vi "UHR-Fleezers Control (host) - Avogadro v1.vi"() -> ()   [LabVIEW 2014] (continued)
          }
          frame True {
          }
        }
        n2943 = local write "Tab Control 6"(T57."Imaging" ("Tab Control 6")) -> ()
        n2944 = local read "T3 X (V)"() -> (w5126:dbl)
        n2945 = local write "MCL Scanning"(w5134) -> ()
        n2946 = local read "T3 Y (V)"() -> (w5125:dbl)
        n2947 = local read "AO2"() -> (w5127:dbl)
        n2948 = local read "AO1"() -> (w5128:dbl)
        n2949 = case shown="True" "Center Scan" {
          tunnel: w5139 -> [w5157 w5179]
          tunnel: w5138 -> [w5156 w5178]
          tunnel: [w5155 w5177] -> w5136
          tunnel: [w5154 w5176] -> w5135
          tunnel: [w5149 w5173] -> w5133
          tunnel: [w5150 w5172] -> w5132
          tunnel: w5128 -> [w5147 w5175]
          tunnel: w5127 -> [w5146 w5174]
          tunnel: "Scan trap 3 or Fl?" -> [w5152 w5171]
          tunnel: w5126 -> [w5151 w5164]
          tunnel: w5125 -> [w5148 w5165]
          frame False {
            w5153 = TRUE ("AI to FIFO")
            n2950 = case shown="True" w5152 {
              tunnel: [w5159 w5163] -> w5150
              tunnel: w5151 -> [_ w5163]
              tunnel: [w5160 w5162] -> w5149
              tunnel: w5148 -> [_ w5162]
              tunnel: w5147 -> [w5160 _]
              tunnel: w5146 -> [w5159 _]
              tunnel: [FALSE ("AI to FIFO") TRUE ("AI to FIFO")] -> w5145
              frame False {
              }
              frame True {
              }
            }
            n2951 = xnode "Read/Write Control"("FPGA VI Reference In"=w5157, "error in"=w5156, "AI to FIFO"=w5153, "APD to FIFO"=w5153, "Start scan (MCL)"=w5153, "ScanTrap 3 or Fl-laser"=w5145) -> ("FPGA VI Reference Out"=w5155:T41, "error out"=w5154:errorcluster)
          }
          frame True {
            n2952 = local read "Actual MCL Inc (V)"() -> (w5166:dbl)
            n2953 = local read "Scan steps (MCL)"() -> (w5167:u64)
            n2954 = local read "Scan lines (y)"() -> (w5168:u64)
            n2955 = local read "Fast Scan Dir"() -> (w5169:bool)
            n2956 = local read "2D or 1D Scan"() -> (w5170:bool)
            n2957 = case shown="True" w5171 {
              tunnel: w5179 -> [w5197 w5215]
              tunnel: w5178 -> [w5196 w5214]
              tunnel: [w5195 w5213] -> w5177
              tunnel: [w5194 w5212] -> w5176
              tunnel: w5175 -> [w5190 _]
              tunnel: w5174 -> [w5189 _]
              tunnel: [w5187 w5207] -> w5173
              tunnel: [w5186 w5206] -> w5172
              tunnel: w5170 -> [w5185 w5205]
              tunnel: w5169 -> [w5184 w5204]
              tunnel: w5168 -> [w5183 w5203]
              tunnel: w5167 -> [w5182 w5202]
              tunnel: w5166 -> [w5180 w5200]
              tunnel: w5165 -> [_ w5199]
              tunnel: w5164 -> [_ w5198]
              frame False {
                w5193 = TRUE ("AI to FIFO")
                n2958 = Bundle("Actual MCL Inc (V)"=w5180, "Scan steps (MCL)"=w5182, "Scan lines (y)"=w5183, "AO1"=w5190, "AO2"=w5189) -> (w5188:T61)  [unwired: 1 in]
                n2959 = call "Center Scan calculation.vi"("2D or 1D Scan"=w5185, "Fast Scan Dir"=w5184, "Input parameters"=w5188) -> ("X"=w5186:dbl, "Y"=w5187:dbl)
                n2960 = call "Volt to I16.vi"("Voltage In"=w5187) -> ("I16 Voltage Out"=w5192:i16)
                n2961 = call "Volt to I16.vi"("Voltage In"=w5186) -> ("I16 Voltage Out"=w5191:i16)
                n2962 = xnode "Read/Write Control"("FPGA VI Reference In"=w5197, "error in"=w5196, "AI to FIFO"=w5193, "APD to FIFO"=w5193, "Start scan (MCL)"=w5193, "AO1 (Y)"=w5192, "AO2 (X)"=w5191, "ScanTrap 3 or Fl-laser"=FALSE ("AI to FIFO")) -> ("FPGA VI Reference Out"=w5195:T41, "error out"=w5194:errorcluster)
              }
              frame True {
                w5211 = TRUE ("AI to FIFO")
                n2963 = Bundle("Actual MCL Inc (V)"=w5200, "Scan steps (MCL)"=w5202, "Scan lines (y)"=w5203, "T3 Y (V)"=w5199, "T3 X (V)"=w5198) -> (w5208:T62)  [unwired: 1 in]
                n2964 = call "Center Scan calculation.vi"("2D or 1D Scan"=w5205, "Fast Scan Dir"=w5204, "Input parameters"=w5208) -> ("X"=w5206:dbl, "Y"=w5207:dbl)
                n2965 = call "Volt to I16.vi"("Voltage In"=w5207) -> ("I16 Voltage Out"=w5210:i16)
                n2966 = call "Volt to I16.vi"("Voltage In"=w5206) -> ("I16 Voltage Out"=w5209:i16)
                n2967 = xnode "Read/Write Control"("FPGA VI Reference In"=w5215, "error in"=w5214, "AI to FIFO"=w5211, "APD to FIFO"=w5211, "Start scan (MCL)"=w5211, "Piezo Trap Y (AO4)"=w5210, "Piezo Trap X (AO5)"=w5209, "ScanTrap 3 or Fl-laser"=TRUE ("AI to FIFO")) -> ("FPGA VI Reference Out"=w5213:T41, "error out"=w5212:errorcluster)
              }
            }
          }
        }
        "Initial Y" <- w5133
        "Initial X" <- w5132
        "wait to reset values" <- w5134
      }
    }
    n2968 = xnode "Read/Write Control"("FPGA VI Reference In"=w4292) -> ("FPGA VI Reference Out"=w4251:T41, "BD1 Frequency Out 1"=w4294:u64)  [unwired: 1 in, 1 out]
    n2969 = And(x="Save scans", y=w4534) -> (x .and. y?=w4554:bool)
    n2970 = call "IR AOM word to freq.vi"("Frequency Word In (U64)"=w4294) -> ("Frequency Out (MHz)"=w4293:dbl)
    n2971 = local read "BD 1 Frequency 2 (MHz)"() -> (w4335:dbl)
    n2972 = Subtract(x=w4335, y=w4293) -> (x-y=w4328:dbl)
    "Current deltaF (MHz)" <- w4328
    n2973 = control-ref of="Piezo trap cursor control"() -> (w4252:refnum<vi>)
    n2974 = Unbundle By Name("Cursor control") -> ("X"=w4254:bool, "Y"=w4253:bool)
    n2975 = local read "APD Elements/DMA read"() -> (w4391:u32)
    n2976 = local read "Trap AI Elements/DMA read"() -> (w4521:u32)
    n2977 = case shown="False" w4254 {
      tunnel: w4252 -> [w4608 w4618]
      tunnel: w4251 -> [_ w4610]
      frame False {
        n2978 = local read "T3 X (V)"() -> (w4609:dbl)
        n2979 = property class="XYGraph (strict)"(reference=w4608, "Cursor.Cursor X"=w4609) -> ()  [unwired: 1 in, 2 out]
      }
      frame True {
        n2980 = property class="XYGraph (strict)"(reference=w4618) -> ("Cursor.Cursor X"=w4615:dbl)  [unwired: 1 in, 2 out]
        n2981 = In Range and Coerce(upper limit=10.0, x=w4615, lower limit=0.0) -> (coerced(x)=w4613:dbl)  [unwired: 1 out]
        n2982 = Multiply(x=3276.7, y=w4613) -> (x*y=w4612:dbl)
        n2983 = To Unsigned Word Integer(number=w4612) -> (unsigned 16bit integer=w4611:u16)
        n2984 = xnode "Read/Write Control"("FPGA VI Reference In"=w4610, "Piezo Trap X (AO5)"=w4611) -> ()  [unwired: 1 in, 2 out]
      }
    }
    n2985 = case shown="False" w4253 {
      tunnel: w4252 -> [w4595 w4607]
      tunnel: w4251 -> [_ w4598]
      frame False {
        n2986 = local read "T3 Y (V)"() -> (w4597:dbl)
        n2987 = Negate(x=w4597) -> (-x=w4596:dbl)
        n2988 = property class="XYGraph (strict)"(reference=w4595, "Cursor.Cursor Y"=w4596) -> ()  [unwired: 1 in, 2 out]
      }
      frame True {
        n2989 = property class="XYGraph (strict)"(reference=w4607) -> ("Cursor.Cursor Y"=w4604:dbl)  [unwired: 1 in, 2 out]
        n2990 = In Range and Coerce(upper limit=0.0, x=w4604, lower limit=-10.0) -> (coerced(x)=w4603:dbl)  [unwired: 1 out]
        n2991 = Negate(x=w4603) -> (-x=w4601:dbl)
        n2992 = Multiply(x=3276.7, y=w4601) -> (x*y=w4600:dbl)
        n2993 = To Unsigned Word Integer(number=w4600) -> (unsigned 16bit integer=w4599:u16)
        n2994 = xnode "Read/Write Control"("FPGA VI Reference In"=w4598, "Piezo Trap Y (AO4)"=w4599) -> ()  [unwired: 1 in, 2 out]
      }
    }
    n2995 = local read "Trap Pos Elements/DMA read"() -> (w4482:u32)
    n2996 = local read "DMA Update Period (s)"() -> (w4313:dbl)
    n2997 = xnode "Invoke Method"("FPGA VI Reference In"=w4486, "error in"=w4485, "Number of Elements"=w4482, "Timeout (ms)"=-1) -> ("Data"=w4454:u16[], "Elements Remaining"=→"Trap Pos FIFO El Remaining":u32)  [unwired: 2 out]
    n2998 = xnode "Get Trap Data"("FPGA VI Reference In"=w4486, "error in"=w4485, "Number of Elements"=w4521, "Timeout (ms)"=-1 ("Timeout")) -> ("FPGA VI Reference Out"=w4334:T41, "error out"=w4424:errorcluster, "Data"=w4317:i16[], "Elements Remaining"=w4588:u32)
    "FIFO El. Rem." <- w4588
    n2999 = local read "Trap AI FIFO Depth"() -> (w4590:u32)
    n3000 = xnode "Get APD Data"("FPGA VI Reference In"=w4486, "error in"=w4485, "Number of Elements"=w4391, "Timeout (ms)"=-1) -> ("Data"=w4307:u32[], "Elements Remaining"=→"APD FIFO Elements Remaining":u32)  [unwired: 2 out]
    n3001 = feedback #1(0.0) -> (w4477:dbl)
    n3002 = To Time Stamp(1:w4477) -> (0:w4290:timestamp)
    n3003 = Add(x=w4313, y=w4477) -> (x+y=w4565:dbl)
    n3004 = feedback-in #1(w4565) -> ()
    n3005 = Subtract(x=w4590, y=w4521) -> (x-y=w4589:u32)
    n3006 = local read "APD Integration Time (s)"() -> (w4299:dbl)
    n3007 = Divide(x=w4588, y=w4589) -> (x/y=w4587:dbl)
    "Buffer Status" <- w4587
    n3008 = local read "Trap Sets"() -> (w4318:u32)
    n3009 = Equal?(x=w4587, y=1.0) -> (x = y?=w4585:bool)
    n3010 = local read "Number of APDs"() -> (w4306:u8)
    n3011 = Decimate 1D Array(w4454) -> (w4451:u16[], w4453:u16[], w4452:u16[], w4297:u16[], w4295:u16[])
    n3012 = case "Alert buffer overflow" shown="True" w4585 {
      frame False {
      }
      frame True {
        n3013 = call <vilib>:"Beep.vi"() -> ()  [unwired: 3 in, 9 out]
        "Overflow (data lost)" <- TRUE ("Overflow (data lost)")
      }
    }
    n3014 = To Unsigned Long Integer(number=w4451) -> (unsigned 32bit integer=w4450:u32[])
    n3015 = Join Numbers(hi=w4453, lo=w4452) -> ((hi.lo)=w4449:u32[])
    n3016 = Divide(x=w4297, y=w4296) -> (x/y=w4278:dbl[])
    n3017 = Divide(x=w4295, y=w4296) -> (x/y=w4277:dbl[])
    n3018 = call "deinterlace.vi"("Detector type"="Detector Type", "Data"=w4317, "Trap sets"=w4318, "Flip x sign"="Flip X Sign") -> ("Channel pattern"=w4314:i32, "Channel names"=w4250:string[], "Deinterlaced normalized data"=w4311:dbl[][], "Deinterlaced data"=w4315:i16[])
    "AI labels" <- w4250
    n3019 = Join Numbers(hi=w4450, lo=w4449) -> ((hi.lo)=w4444:u64[])
    n3020 = local read "Data Period (s)"() -> (w4284:dbl)
    n3021 = call "APD data extraction.vi"("Data"=w4307, "Number of APD's"=w4306, "APD integration time (s)"=w4299, "APD Ave N"="APD Ave N", "APD Disp. Downsample"="APD Disp. Downsample", "APD Disp. Scale"="APD Disp. Scale", "Time Stamp"=w4290) -> ("Output cluster"=→"APD rates cluster":T1, "Output Data"=w4302:T63, "Output waveform"=w4301:waveform(dbl)[], "APD Display period (s)"=w4300:dbl)
    "APD Display Period (s)" <- w4300
    n3022 = call "IR AOM word to freq - vec.vi"("Frequency Word In (double vec)"=w4444) -> ("Frequency Out"=w4481:dbl[])
    n3023 = Decimate 1D Array(w4277) -> (w4274:dbl[], w4273:dbl[])
    n3024 = Decimate 1D Array(w4278) -> (w4276:dbl[], w4275:dbl[])
    n3025 = Add(x=w4276, y=w4275) -> (x+y=w4272:dbl[])
    n3026 = Add(x=w4274, y=w4273) -> (x+y=w4271:dbl[])
    n3027 = Decimate 1D Array(w4481) -> (w4480:dbl[], w4479:dbl[])
    n3028 = Divide(x=w4272, y=w4270) -> (x/y=w4268:dbl[])
    n3029 = Divide(x=w4271, y=w4270) -> (x/y=w4269:dbl[])
    n3030 = Reciprocal(x=w4300) -> (1/x=→"APD Display Freq. (Hz)":dbl)
    n3031 = Build Array(w4480, w4479, w4268, w4269) -> (w4291:dbl[][])
    n3032 = Multiply(x=w4284, y="Trap Disp. Downsample") -> (x*y=w4478:dbl)
    "Display Period (s)" <- w4478
    n3033 = for {
      tunnel: w4311 -> [w4633] mode=indexing
      tunnel: [w4632] -> w4249 mode=indexing
      n3034 = call-poly <vilib>:"Mean.vi"("X"=w4633) -> ("mean"=w4632:dbl)  [unwired: 1 out]
    }
    "Values" <- w4249
    n3035 = call "Generate Waveform.vi"("Downsampling"="Trap Disp. Downsample", "Data Period (s)"=w4284, "Data"=w4311, "Plot names"=w4250, "Time Stamp"=w4290) -> ("Downsampled data"=w4309:waveform(dbl)[], "Non downsampled waveform"=w4308:waveform(dbl)[])
    n3036 = Multiply(x="APD Disp. Scale", y=w4301) -> (x*y=w4499:waveform(dbl)[])
    n3037 = Reciprocal(x=w4478) -> (1/x=→"Trap Disp. Freq. (Hz)":dbl)
    n3038 = Multiply(x="APD Disp. Downsample", y=w4299) -> (x*y=w4498:dbl)
    n3039 = Decimate 1D Array(w4315) -> (w4469:i16[], w4468:i16[], w4466:i16[], w4465:i16[])  [unwired: 9 out]
    n3040 = Divide(x=w4499, y=w4498) -> (x/y=w4396:waveform(dbl)[])
    n3041 = case shown="1" "Plot Trap Positions" {
      tunnel: [w4619 w4627] -> w4285
      frame 0, Default {
        n3042 = local read "BD 1 Frequency 2 (MHz)"() -> (w4622:dbl)
        n3043 = local read "BD 1 Frequency 1 (MHz)"() -> (w4623:dbl)
        n3044 = local read "T3 Y (V)"() -> (w4620:dbl)
        n3045 = local read "T3 X (V)"() -> (w4621:dbl)
        n3046 = Build Array(w4623, w4622, w4621, w4620) -> (w4619:dbl[])
      }
      frame 1 {
        w4626 = 60.0
        n3047 = Build Array(w4626, w4626, "Piezo trap x\noffset (V)", "Piezo trap y\noffset (V)") -> (w4627:dbl[])
      }
    }
    n3048 = Divide(x=w4469, y=w4468) -> (x/y=w4470:dbl[])
    n3049 = Divide(x=w4466, y=w4465) -> (x/y=w4467:dbl[])
    n3050 = local read "AOM X Cal (nm/MHz)"() -> (w4287:dbl)
    n3051 = Split 1D Array(array=w4470, index="N El. to Ave.") -> (second subarray=w4473:dbl[])  [unwired: 1 out]
    n3052 = Split 1D Array(array=w4467, index="N El. to Ave.") -> (second subarray=w4472:dbl[])  [unwired: 1 out]
    n3053 = Index Array(array=w4396, index=0) -> (element=w4494:waveform(dbl))
    n3054 = Index Array(array=w4396, index=1) -> (element=w4492:waveform(dbl))
    n3055 = Index Array(array=w4396, index=2) -> (element=w4398:waveform(dbl))
    n3056 = call-poly <vilib>:"Mean.vi"("X"=w4473) -> ("mean"=w4461:dbl)  [unwired: 1 out]
    n3057 = call-poly <vilib>:"Mean.vi"("X"=w4472) -> ("mean"=w4460:dbl)  [unwired: 1 out]
    n3058 = Subtract(x=w4494, y="APD 1 Offset") -> (x-y=w4490:waveform(dbl))
    n3059 = Subtract(x=w4492, y="APD 2 Offset") -> (x-y=w4489:waveform(dbl))
    n3060 = Subtract(x=w4398, y="APD 3 Offset") -> (x-y=w4395:waveform(dbl))
    n3061 = Build Array(w4490, w4489, w4395) -> (→"APD Chart":waveform(dbl)[])
    n3062 = Build Array(w4287, w4287, "Piezo Trap X cal (nm/V)", "Piezo Trap Y cal (nm/V)") -> (w4286:dbl[])
    n3063 = local read "Trap X AI1 (DMA)"() -> (w4471:T19)
    n3064 = To Fixed-Point(number=w4460) -> (fixed-point=w4458:fxp<+/-,16,1>)  [unwired: 1 in]
    n3065 = To Fixed-Point(number=w4461) -> (fixed-point=w4459:fxp<+/-,16,1>)  [unwired: 1 in]
    n3066 = Cluster To Array(cluster="Negate Axis") -> (array=w4279:bool[])
    n3067 = call "Generate Trap Positiion Waveform.vi"("Base trap positions"=w4285, "Data Period (s)"=w4284, "Input data"=w4291, "Position calibration values"=w4286, "Trap Pos. Disp. Downsample (s)"="Trap Pos. Disp. Downsample", "Negate axis"=w4279, "Time Stamp"=w4290) -> ("Output waveforms"=w4256:waveform(dbl)[], "Output position arrays"=w4248:cluster{"X":dbl[], "Y":dbl[]}[])  [unwired: 2 in]
    "Trap Positions" <- w4256
    n3068 = Bundle By Name(cluster=w4471, "Set 1"=w4459, "Set 2"=w4458) -> (→"Trap X AI1 (DMA)":T19)
    n3069 = Initialize Array(0.0) -> (w4281:dbl[][])  [unwired: 2 in]
    n3070 = local read "Display Period (s)"() -> (w4508:dbl)
    n3071 = for {
      tunnel: w4256 -> [w4631] mode=indexing
      shift-right: [w4629] -> w4258
      shift-left: w4281 -> [w4630]
      n3072 = Unbundle By Name(w4631) -> ("Y"=w4628:dbl[])
      n3073 = Build Array (concatenate)(w4630, w4628) -> (w4629:dbl[][])
    }
    n3074 = Build Array (concatenate)(w4301, w4309) -> (w4312:waveform(dbl)[])
    "All Signals" <- w4312
    n3075 = flat-sequence {
      tunnel: w4248 -> [w4594]
      frame #0 {
        "Positions \nand displacements" <- w4594
      }
      frame #1 {
      }
    }
    n3076 = Divide(x="Bead Sep. Int. Time (s)", y=w4508) -> (x/y=w4264:dbl)
    n3077 = feedback #2(w4258) -> (w4265:dbl[][])
    n3078 = call "Trap Pos RMS.vi"("Accumulated array"=w4265, "New Array"=w4258, "Number of sets to average"=w4264) -> ("Output accumulated array"=w4263:dbl[][], "RMS"=w4261:dbl[], "Mean"=w4262:dbl[])
    n3079 = feedback-in #2(w4263) -> ()
    n3080 = Index Array(array=w4258, index (row)=0 ("index")) -> (element=w4257:dbl[])  [unwired: 1 in]
    n3081 = Array To Cluster(array=w4261) -> (cluster=→"Trap RMS (ang)":T64)
    n3082 = Array To Cluster(array=w4262) -> (cluster=→"Mean Trap Positions (nm)":T65)
    n3083 = local read "Data points/scans (MCL)"() -> (w4548:dbl)
    n3084 = Unbundle(w4302) -> ("APD 1"=w4394:u32[])  [unwired: 2 out]
    n3085 = To Double Precision Float(number=w4394) -> (double precision float=w4516:dbl[])
    n3086 = Increment(x=w4548) -> (x+1=w4549:dbl)
    n3087 = feedback #3(w4549) -> (w4552:dbl)
    n3088 = Select(t=0, s=w4539, f=w4552) -> (s? t:f=w4545:dbl)
    n3089 = Array Size(array=w4516) -> (size(s)=w4551:i32)
    n3090 = Add(x=w4551, y=w4545) -> (x+y=w4546:dbl)
    n3091 = Greater?(x=w4546, y=w4548) -> (0:w4547:bool)
    n3092 = local read "MCL Scanning"() -> (w4542:bool)
    n3093 = Select(t=w4545, s=w4547, f=w4546) -> (s? t:f=w4544:dbl)
    n3094 = feedback-in #3(w4544) -> ()
    n3095 = Index Array(array=w4309, index="index 1") -> (element=w4386:waveform(dbl))
    n3096 = Index Array(array=w4309, index="index 2") -> (element=w4390:waveform(dbl))
    n3097 = Unbundle By Name(w4386) -> ("Y"=w4385:dbl[])
    n3098 = Unbundle By Name(w4390) -> ("Y"=w4389:dbl[])
    n3099 = Not(x=w4547) -> (.not. x?=w4541:bool)
    n3100 = And(x=w4541, y=w4542) -> (x .and. y?=w4543:bool)
    n3101 = call-poly <vilib>:"Mean.vi"("X"=w4385) -> ("mean"=→"Trap 1 sum mean":dbl)  [unwired: 1 out]
    n3102 = call-poly <vilib>:"Mean.vi"("X"=w4389) -> ("mean"=→"Trap 2 sum mean":dbl)  [unwired: 1 out]
    n3103 = Or(x=w4543, y=w4539) -> (x .or. y?=w4540:bool)
    n3104 = Equal?(x="Tab Control 6", y=T53."High Res Display") -> (x = y?=w4518:bool)
    n3105 = case shown="True" "X or Y?" {
      tunnel: w4309 -> [w4742 w4748]
      tunnel: [w4743 w4747] -> w4361
      tunnel: [w4741 w4746] -> w4358
      frame False {
        n3106 = Index Array(array=w4742, index=0) -> (element=w4743:waveform(dbl))
        n3107 = Index Array(array=w4742, index=3) -> (element=w4741:waveform(dbl))
      }
      frame True {
        n3108 = Index Array(array=w4748, index=1) -> (element=w4747:waveform(dbl))
        n3109 = Index Array(array=w4748, index=4) -> (element=w4746:waveform(dbl))
      }
    }
    n3110 = case "For displaying the high resolution display (no downsampling)" shown="True" w4518 {
      tunnel: w4308 -> [_ w4881]
      frame False {
      }
      frame True {
        n3111 = Index Array(array=w4881, index="High Res. Display") -> (element=w4882:waveform(dbl))
        n3112 = call <vilib>:"Std Deviation and Variance.vi"("X"=w4882) -> ("mean"=w4889:dbl, "standard deviation"=w4894:dbl)  [unwired: 1 in, 1 out]
        "Mean Intensity" <- w4889
        "Sigma" <- w4894
        n3113 = Subtract(x=w4882, y=w4889) -> (x-y=w4888:waveform(dbl))
        n3114 = Select(t=w4888, s="Subtract mean", f=w4882) -> (s? t:f=→"1 Channel":waveform(dbl))
        n3115 = Divide(x=w4894, y=w4889) -> (x/y=→"Sigma/Mean":dbl)
        n3116 = feedback #4(1) -> (w4883:i32)
        n3117 = Greater Or Equal?(x=w4883, y="Slow mean N ave.") -> (x >= y?=w4896:bool)
        n3118 = Increment(x=w4883) -> (x+1=w4898:i32)
        n3119 = Select(t=1, s=w4896, f=w4898) -> (s? t:f=w4885:i32)
        n3120 = feedback-in #4(w4885) -> ()
        n3121 = feedback #5() -> (w4886:waveform(dbl))  [unwired: 1 out]
        n3122 = case shown="Default" w4883 {
          tunnel: [w4901 w4904] -> w4887
          tunnel: w4886 -> [w4903 _]
          tunnel: w4882 -> [w4902 w4904]
          frame Default {
            n3123 = call-poly <vilib>:"Append Waveforms.vi"("waveform B"=w4902, "waveform A"=w4903) -> ("waveform out"=w4901:waveform(dbl))  [unwired: 1 in, 8 out]
          }
          frame 1 {
          }
        }
        n3124 = feedback-in #5(w4887) -> ()
        n3125 = case shown="True" w4896 {
          tunnel: w4887 -> [_ w4900]
          frame False {
          }
          frame True {
            n3126 = call-poly <vilib>:"Mean.vi"("X"=w4900) -> ("mean"=→"Slow mean":dbl)  [unwired: 1 out]
          }
        }
      }
    }
    n3127 = case "For plotting results of scanning MCL (fluorescence and detection laser images)" shown="True" w4540 {
      tunnel: w4539 -> [_ w4983]
      tunnel: w4548 -> [_ _]
      tunnel: w4308 -> [_ w5079]
      tunnel: w4487 -> [_ w5011]
      tunnel: w4302 -> [_ w4989]
      frame False {
      }
      frame True {
        w4952 = u32 0 items=["Horizontal", "Vertical", "Central", "1st Diagonal", "2nd Diagonal"] ("Type of Symmetry")
        w4956 = u32 0 items=["Horizontal", "Vertical", "Central", "1st Diagonal", "2nd Diagonal"] ("Type of Symmetry")
        w4957 = u32 0 items=["Horizontal", "Vertical", "Central", "1st Diagonal", "2nd Diagonal"] ("Type of Symmetry")
        w4958 = u32 0 items=["Horizontal", "Vertical", "Central", "1st Diagonal", "2nd Diagonal"] ("Type of Symmetry")
        w4962 = u32 0 items=["Horizontal", "Vertical", "Central", "1st Diagonal", "2nd Diagonal"] ("Type of Symmetry")
        # "Modified by Ronen \nbecause we do not have\nthe license for the\ntwo last image \nmanipulation VI's"
        n3128 = local read "Scan trap 3 or Fl?"() -> (w4943:bool)
        n3129 = case shown="True" w4943 {
          tunnel: [10 ("index") 0 ("index")] -> w5086
          tunnel: [11 ("index") 1 ("index")] -> w5083
          frame False {
          }
          frame True {
          }
        }
        n3130 = Unbundle(w4989) -> ("APD 1"=w4988:u32[], "APD 2"=w4986:u32[], "APD 3"=w4984:u32[])
        n3131 = To Double Precision Float(number=w4988) -> (double precision float=w4987:dbl[])
        n3132 = To Double Precision Float(number=w4986) -> (double precision float=w4985:dbl[])
        n3133 = To Double Precision Float(number=w4984) -> (double precision float=w4977:dbl[])
        n3134 = Index Array(array=w5079, index=w5086) -> (element=w5085:waveform(dbl))
        n3135 = Index Array(array=w5079, index=w5083) -> (element=w5082:waveform(dbl))
        n3136 = local read "Cycles/step (MCL)"() -> (w5041:u64)
        n3137 = Index Array(array=w5079, index="Channel") -> (element=w5081:waveform(dbl))
        n3138 = Unbundle(w5011) -> ("New Image"=w5010:T7, "New Image"=w5009:T7, "New Image"=w4990:T7, "New Image"=w4991:T7, "New Image"=w4992:T7)
        n3139 = local read "Scan steps (MCL)"() -> (w4979:u64)
        n3140 = Unbundle By Name(w5085) -> ("Y"=w5043:dbl[])
        n3141 = Unbundle By Name(w5082) -> ("Y"=w5045:dbl[])
        n3142 = local read "Scan lines (y)"() -> (w4980:u64)
        n3143 = local read "N APD Samp/step"() -> (w4982:dbl)
        n3144 = Unbundle By Name(w5081) -> ("Y"=w5050:dbl[])
        n3145 = call "downsample 1D array - double.vi"("Ave N"=w5041, "Array In"=w5043) -> ("Array Out"=w5042:dbl[])  [unwired: 1 out]
        n3146 = call "downsample 1D array - double.vi"("Ave N"=w5041, "Array In"=w5045) -> ("Array Out"=w5044:dbl[])  [unwired: 1 out]
        n3147 = call "downsample 1D array - double.vi"("Ave N"=w5041, "Array In"=w5050) -> ("Array Out"=w5049:dbl[])  [unwired: 1 out]
        n3148 = Multiply(x=w4979, y=u64 2) -> (x*y=w4981:u64)
        n3149 = feedback #6(w4985) -> (w5029:dbl[])
        n3150 = Build Array (concatenate)(w5029, w4985) -> (w5028:dbl[])
        n3151 = feedback #7(w4977) -> (w4978:dbl[])
        n3152 = Build Array (concatenate)(w4978, w4977) -> (w4976:dbl[])
        n3153 = Select(t=w4985, s=w4983, f=w5028) -> (s? t:f=w5013:dbl[])
        n3154 = feedback-in #6(w5013) -> ()
        n3155 = Select(t=w4977, s=w4983, f=w4976) -> (s? t:f=w4994:dbl[])
        n3156 = feedback-in #7(w4994) -> ()
        n3157 = feedback #8(w4987) -> (w5104:dbl[])
        n3158 = Build Array (concatenate)(w5104, w4987) -> (w5087:dbl[])
        n3159 = Select(t=w4987, s=w4983, f=w5087) -> (s? t:f=w5091:dbl[])
        n3160 = feedback-in #8(w5091) -> ()
        n3161 = feedback #9(w5042) -> (w5093:dbl[])
        n3162 = Build Array (concatenate)(w5093, w5042) -> (w5084:dbl[])
        n3163 = feedback #10(w5049) -> (w5102:dbl[])
        n3164 = Build Array (concatenate)(w5102, w5049) -> (w5101:dbl[])
        n3165 = feedback #11(w5044) -> (w5095:dbl[])
        n3166 = Build Array (concatenate)(w5095, w5044) -> (w5096:dbl[])
        n3167 = Select(t=w5042, s=w4983, f=w5084) -> (s? t:f=w5046:dbl[])
        n3168 = feedback-in #9(w5046) -> ()
        n3169 = Select(t=w5049, s=w4983, f=w5101) -> (s? t:f=w5048:dbl[])
        n3170 = feedback-in #10(w5048) -> ()
        n3171 = Select(t=w5044, s=w4983, f=w5096) -> (s? t:f=w5047:dbl[])
        n3172 = feedback-in #11(w5047) -> ()
        n3173 = call "integrate 1D array interval - double.vi"("Ave N"=w4982, "Array In"=w5013) -> ("Array Out"=w5024:dbl[])  [unwired: 1 out]
        n3174 = call "integrate 1D array interval - double.vi"("Ave N"=w4982, "Array In"=w4994) -> ("Array Out"=w5005:dbl[])  [unwired: 1 out]
        n3175 = call "integrate 1D array interval - double.vi"("Ave N"=w4982, "Array In"=w5091) -> ("Array Out"=w5090:dbl[])  [unwired: 1 out]
        n3176 = Array Size(array=w5024) -> (size(s)=w5025:i32)
        n3177 = Array Size(array=w5005) -> (size(s)=w5006:i32)
        n3178 = Array Size(array=w5090) -> (size(s)=w5092:i32)
        n3179 = Multiply(x=w4980, y=w4981) -> (x*y=w5027:u64)
        n3180 = Multiply(x=w4980, y=w4981) -> (x*y=w5008:u64)
        n3181 = Multiply(x=w4980, y=w4981) -> (x*y=w5100:u64)
        n3182 = Subtract(x=w5027, y=w5025) -> (x-y=w5018:u64)
        n3183 = call-poly <vilib>:"Mean.vi"("X"=w5024) -> ("mean"=w5015:dbl)  [unwired: 1 out]
        n3184 = Subtract(x=w5008, y=w5006) -> (x-y=w4999:u64)
        n3185 = call-poly <vilib>:"Mean.vi"("X"=w5005) -> ("mean"=w4996:dbl)  [unwired: 1 out]
        n3186 = Subtract(x=w5100, y=w5092) -> (x-y=w5040:u64)
        n3187 = call-poly <vilib>:"Mean.vi"("X"=w5090) -> ("mean"=w5037:dbl)  [unwired: 1 out]
        n3188 = call-poly <vilib>:"Mean.vi"("X"=w5046) -> ("mean"=w5030:dbl)  [unwired: 1 out]
        n3189 = call-poly <vilib>:"Mean.vi"("X"=w5048) -> ("mean"=w5035:dbl)  [unwired: 1 out]
        n3190 = call-poly <vilib>:"Mean.vi"("X"=w5047) -> ("mean"=w5033:dbl)  [unwired: 1 out]
        n3191 = Initialize Array(1.0 ("element"), w5018) -> (w5014:dbl[])
        n3192 = Initialize Array(1.0 ("element"), w4999) -> (w4995:dbl[])
        n3193 = Initialize Array(1.0 ("element"), w5040) -> (w5031:dbl[])
        n3194 = Multiply(x=w5014, y=w5015) -> (x*y=w5016:dbl[])
        n3195 = Multiply(x=w4995, y=w4996) -> (x*y=w4997:dbl[])
        n3196 = Multiply(x=w5031, y=w5037) -> (x*y=w5038:dbl[])
        n3197 = Multiply(x=w5031, y=w5033) -> (x*y=w5034:dbl[])
        n3198 = Multiply(x=w5031, y=w5035) -> (x*y=w5036:dbl[])
        n3199 = Multiply(x=w5031, y=w5030) -> (x*y=w5032:dbl[])
        n3200 = Build Array (concatenate)(w5024, w5016) -> (w5026:dbl[])
        n3201 = Build Array (concatenate)(w5005, w4997) -> (w5007:dbl[])
        n3202 = Build Array (concatenate)(w5090, w5038) -> (w5099:dbl[])
        n3203 = Build Array (concatenate)(w5046, w5032) -> (w5094:dbl[])
        n3204 = Build Array (concatenate)(w5048, w5036) -> (w5098:dbl[])
        n3205 = Build Array (concatenate)(w5047, w5034) -> (w5097:dbl[])
        n3206 = Reshape Array(w5026, w4980, w4981) -> (w5022:dbl[][])
        n3207 = Reshape Array(w5007, w4980, w4981) -> (w5003:dbl[][])
        n3208 = Reshape Array(w5099, w4980, w4981) -> (w5077:dbl[][])
        n3209 = Reshape Array(w5094, w4980, w4981) -> (w5060:dbl[][])
        n3210 = Reshape Array(w5098, w4980, w4981) -> (w5052:dbl[][])
        n3211 = Reshape Array(w5097, w4980, w4981) -> (w5067:dbl[][])
        n3212 = Array Subset(array=w5022, index (col)=0 ("index"), length (col)=w4979) -> (w5021:dbl[][])  [unwired: 2 in]
        n3213 = Array Subset(array=w5022, index (col)=w4979) -> (w5019:dbl[][])  [unwired: 3 in]
        n3214 = Array Subset(array=w5003, index (col)=0 ("index"), length (col)=w4979) -> (w5002:dbl[][])  [unwired: 2 in]
        n3215 = Array Subset(array=w5003, index (col)=w4979) -> (w5000:dbl[][])  [unwired: 3 in]
        n3216 = Array Subset(array=w5067, index (col)=0 ("index"), length (col)=w4979) -> (w5072:dbl[][])  [unwired: 2 in]
        n3217 = Array Subset(array=w5067, index (col)=w4979) -> (w5070:dbl[][])  [unwired: 3 in]
        n3218 = Array Subset(array=w5077, index (col)=0 ("index"), length (col)=w4979) -> (w5076:dbl[][])  [unwired: 2 in]
        n3219 = Array Subset(array=w5077, index (col)=w4979) -> (w5074:dbl[][])  [unwired: 3 in]
        n3220 = Array Subset(array=w5052, index (col)=0 ("index"), length (col)=w4979) -> (w5058:dbl[][])  [unwired: 2 in]
        n3221 = Array Subset(array=w5052, index (col)=w4979) -> (w5056:dbl[][])  [unwired: 3 in]
        n3222 = Array Subset(array=w5060, index (col)=0 ("index"), length (col)=w4979) -> (w5065:dbl[][])  [unwired: 2 in]
        n3223 = Array Subset(array=w5060, index (col)=w4979) -> (w5063:dbl[][])  [unwired: 3 in]
        n3224 = for {
          tunnel: w5021 -> [w5112] mode=indexing
          tunnel: [w5111] -> w5020 mode=indexing
          workers-P: _ -> [_]
          n3225 = Reverse 1D Array(array=w5112) -> (reversed array=w5111:dbl[])
        }
        n3226 = for {
          tunnel: w5002 -> [w5110] mode=indexing
          tunnel: [w5109] -> w5001 mode=indexing
          workers-P: _ -> [_]
          n3227 = Reverse 1D Array(array=w5110) -> (reversed array=w5109:dbl[])
        }
        n3228 = for {
          tunnel: w5072 -> [w5118] mode=indexing
          tunnel: [w5117] -> w5071 mode=indexing
          workers-P: _ -> [_]
          n3229 = Reverse 1D Array(array=w5118) -> (reversed array=w5117:dbl[])
        }
        n3230 = for {
          tunnel: w5076 -> [w5120] mode=indexing
          tunnel: [w5119] -> w5075 mode=indexing
          workers-P: _ -> [_]
          n3231 = Reverse 1D Array(array=w5120) -> (reversed array=w5119:dbl[])
        }
        n3232 = for {
          tunnel: w5058 -> [w5114] mode=indexing
          tunnel: [w5113] -> w5057 mode=indexing
          workers-P: _ -> [_]
          n3233 = Reverse 1D Array(array=w5114) -> (reversed array=w5113:dbl[])
        }
        n3234 = for {
          tunnel: w5065 -> [w5116] mode=indexing
          tunnel: [w5115] -> w5064 mode=indexing
          workers-P: _ -> [_]
          n3235 = Reverse 1D Array(array=w5116) -> (reversed array=w5115:dbl[])
        }
        n3236 = Index Array(array=w5077, index (row)=0) -> (element=→"Waveform Graph":dbl[])  [unwired: 1 in]
        n3237 = Add(x=w5020, y=w5019) -> (x+y=w5012:dbl[][])
        n3238 = Add(x=w5001, y=w5000) -> (x+y=w4993:dbl[][])
        n3239 = Add(x=w5071, y=w5070) -> (x+y=w5069:dbl[][])
        n3240 = Add(x=w5075, y=w5074) -> (x+y=w5051:dbl[][])
        n3241 = Add(x=w5057, y=w5056) -> (x+y=w5055:dbl[][])
        n3242 = Add(x=w5064, y=w5063) -> (x+y=w5062:dbl[][])
        n3243 = Divide(x=w5055, y=2) -> (x/y=w5053:dbl[][])
        n3244 = Divide(x=w5069, y=2) -> (x/y=w4970:dbl[][])
        n3245 = To Single Precision Float(number=w5051) -> (single precision float=w4974:sgl[][])
        n3246 = To Single Precision Float(number=w5012) -> (single precision float=w4969:sgl[][])
        n3247 = To Single Precision Float(number=w4993) -> (single precision float=w4968:sgl[][])
        n3248 = Divide(x=w5062, y=2) -> (x/y=w4971:dbl[][])
        n3249 = Transpose 2D Array(2D array=w5053) -> (transposed array=→"Data map":dbl[][])
        n3250 = To Single Precision Float(number=w4970) -> (single precision float=w4973:sgl[][])
        n3251 = To Single Precision Float(number=w4971) -> (single precision float=w4972:sgl[][])
        n3252 = call "IMAQ ArrayToImage"("Image Pixels (Float)"=w4974, "Image"=w5010) -> ("Image Out"=w4967:T7)  [unwired: 8 in, 1 out]
        n3253 = call "IMAQ ArrayToImage"("Image Pixels (Float)"=w4969, "Image"=w5009) -> ("Image Out"=w4966:T7)  [unwired: 8 in, 1 out]
        n3254 = call "IMAQ ArrayToImage"("Image Pixels (Float)"=w4968, "Image"=w4990) -> ("Image Out"=w4965:T7)  [unwired: 8 in, 1 out]
        n3255 = call "IMAQ ArrayToImage"("Image Pixels (Float)"=w4973, "Image"=w4991) -> ("Image Out"=w4964:T7)  [unwired: 8 in, 1 out]
        n3256 = call "IMAQ ArrayToImage"("Image Pixels (Float)"=w4972, "Image"=w4992) -> ("Image Out"=w4963:T7)  [unwired: 8 in, 1 out]
        n3257 = call "IMAQ Symmetry"("Type of Symmetry"=w4962, "Image Src"=w4967) -> ("Image Dst Out"=w4960:T7)  [unwired: 3 in, 1 out]
        n3258 = call "IMAQ Symmetry"("Type of Symmetry"=w4956, "Image Src"=w4966) -> ("Image Dst Out"=w4954:T7)  [unwired: 3 in, 1 out]
        n3259 = call "IMAQ Symmetry"("Type of Symmetry"=w4952, "Image Src"=w4965) -> ("Image Dst Out"=w4950:T7)  [unwired: 3 in, 1 out]
        n3260 = call "IMAQ Symmetry"("Type of Symmetry"=w4958, "Image Src"=w4964) -> ("Image Dst Out"=→"Detection Laser X":T7)  [unwired: 3 in, 1 out]
        n3261 = call "IMAQ Symmetry"("Type of Symmetry"=w4957, "Image Src"=w4963) -> ("Image Dst Out"=→"Detection Laser Y":T7)  [unwired: 3 in, 1 out]
        n3262 = call "IMAQ Set Simple Calibration"("Calibration Axis Info"=T54 {"Origin Pixel"={"X"=0.0, "Y"=0.0}, "Angle Relative to Horizontal (deg)"=0.0, "Axis Reference"=0}, "Grid Descriptor"=T55 {"X Step"=0.3, "Y Step"=0.3, "Unit"=enum."Undefined"}, "Image"=w4954) -> ("Calibrated Image"=→"APD 2":T7)  [unwired: 7 in, 1 out]
        n3263 = call "IMAQ Set Simple Calibration"("Calibration Axis Info"=T54 {"Origin Pixel"={"X"=0.0, "Y"=0.0}, "Angle Relative to Horizontal (deg)"=0.0, "Axis Reference"=0}, "Grid Descriptor"=T55 {"X Step"=0.3, "Y Step"=0.3, "Unit"=enum."Undefined"}, "Image"=w4950) -> ("Calibrated Image"=→"APD 3":T7)  [unwired: 7 in, 1 out]
        n3264 = call "IMAQ Set Simple Calibration"("Calibration Axis Info"=T54 {"Origin Pixel"={"X"=0.0, "Y"=0.0}, "Angle Relative to Horizontal (deg)"=0.0, "Axis Reference"=0}, "Grid Descriptor"=T55 {"X Step"=0.3, "Y Step"=0.3, "Unit"=enum."Undefined"}, "Image"=w4960) -> ("Calibrated Image"=→"APD 1":T7)  [unwired: 7 in, 1 out]
      }
    }
    n3265 = case "For computing FFTs for display" shown="True" "Compute FFT" {
      tunnel: w4308 -> [_ w5317]
      frame False {
      }
      frame True {
        n3266 = Build Array("FFT 1 Choice 1", "FFT 1 Choice 2", "FFT 2 Choice 1", "FFT 2 Choice 2") -> (w5310:u16[])
        n3267 = Array Size(array=w5317) -> (size(s)=w5316:i32)
        n3268 = feedback-in #12(w5310) -> ()
        n3269 = feedback #12(u16[] [100, 100, 100, 100]) -> (w5311:u16[])
        n3270 = feedback-in #13("# Spectra to Ave.") -> ()
        n3271 = feedback #13("# Spectra to Ave.") -> (w5308:dbl)
        n3272 = Not Equal?(x="# Spectra to Ave.", y=w5308) -> (x != y?=w5307:bool)
        n3273 = Not Equal?(x=w5310, y=w5311) -> (x != y?=w5309:bool)
        n3274 = feedback #14(1.0) -> (w5294:dbl)
        n3275 = Compound Arithmetic op=OR("Reset FFT", w5309, w5307) -> (w5292:bool)
        n3276 = Select(t=1.0, s=w5292, f=w5294) -> (s? t:f=w5296:dbl)
        n3277 = Greater?(x=w5296, y="# Spectra to Ave.") -> (0:w5315:bool)
        n3278 = Increment(x=w5296) -> (x+1=w5295:dbl)
        n3279 = feedback-in #14(w5295) -> ()
        n3280 = local read "DMA Update Period (s)"() -> (w5290:dbl)
        n3281 = Multiply(x="# Spectra to Ave.", y=w5290) -> (x*y=→"Ave. Time (s)":dbl)
        n3282 = Build Array(cluster{"f0":dbl, "df":dbl, "magnitude":dbl[]} {"f0"=0.0, "df"=0.0, "magnitude"=[]} ("PSD")) -> (w5299:cluster{"f0":dbl, "df":dbl, "magnitude":dbl[]}[])
        n3283 = Build Array(w5299, w5299, w5299, w5299) -> (w5301:T66)
        n3284 = feedback #15(w5301) -> (w5306:T66)
        n3285 = for {
          N: 4 -> [_]
          tunnel: w5310 -> [w5339] mode=indexing
          tunnel: w5317 -> [w5340]
          tunnel: w5316 -> [w5342]
          tunnel: w5292 -> [w5335]
          tunnel: w5315 -> [w5334]
          tunnel: "# Spectra to Ave." -> [w5333]
          tunnel: [w5332] -> w5305 mode=indexing
          tunnel: w5306 -> [w5337] mode=indexing
          tunnel: [w5336] -> w5293 mode=indexing
          tunnel: w5296 -> [w5331]
          n3286 = Less?(x=w5339, y=w5342) -> (x < y?=w5341:bool)
          n3287 = Index Array(array=w5340, index=w5339) -> (element=w5338:waveform(dbl))
          n3288 = case shown="True" w5341 {
            tunnel: w5338 -> [_ w5359]
            tunnel: w5337 -> [w5344 w5357]
            tunnel: [w5344 w5345] -> w5336
            tunnel: w5335 -> [_ w5356]
            tunnel: w5334 -> [_ w5349]
            tunnel: w5333 -> [_ w5348]
            tunnel: [cluster{"f0":dbl, "df":dbl, "magnitude":dbl[]} {"f0"=0.0, "df"=0.0, "magnitude"=[]} ("PSD") w5350] -> w5332
            tunnel: w5331 -> [_ w5347]
            frame False {
            }
            frame True {
              n3289 = call <vilib>:"Std Deviation and Variance.vi"("X"=w5359) -> ("mean"=w5360:dbl)  [unwired: 1 in, 2 out]
              n3290 = Subtract(x=w5359, y=w5360) -> (x-y=w5358:waveform(dbl))
              n3291 = xnode "Spectral Measurements"("Signals"=w5358) -> ("PSD"=w5352:cluster{"f0":dbl, "df":dbl, "magnitude":dbl[]})  [unwired: 1 in, 1 out]
              n3292 = case shown="False" w5356 {
                tunnel: w5357 -> [w5369 _]
                tunnel: [w5365 w5374] -> w5345
                tunnel: w5352 -> [w5368 w5375]
                tunnel: w5349 -> [w5367 _]
                frame False {
                  n3293 = Build Array (concatenate)(w5369, w5368) -> (w5366:cluster{"f0":dbl, "df":dbl, "magnitude":dbl[]}[])
                  n3294 = case shown="True" w5367 {
                    tunnel: w5366 -> [w5370 w5373]
                    tunnel: [w5370 w5371] -> w5365
                    frame False {
                    }
                    frame True {
                      n3295 = Delete From Array(array=w5373, index=0) -> (array with subset deleted=w5371:cluster{"f0":dbl, "df":dbl, "magnitude":dbl[]}[])  [unwired: 1 in, 1 out]
                    }
                  }
                }
                frame True {
                  n3296 = Build Array(w5375) -> (w5374:cluster{"f0":dbl, "df":dbl, "magnitude":dbl[]}[])
                }
              }
              n3297 = for {
                tunnel: w5345 -> [w5364] mode=indexing
                tunnel: [w5363] -> w5355 mode=indexing
                workers-P: _ -> [_]
                n3298 = Unbundle By Name(w5364) -> ("magnitude"=w5363:dbl[])
              }
              n3299 = Transpose 2D Array(2D array=w5355) -> (transposed array=w5354:dbl[][])
              n3300 = for {
                tunnel: w5354 -> [w5362] mode=indexing
                tunnel: [w5361] -> w5353 mode=indexing
                workers-P: _ -> [_]
                n3301 = Add Array Elements(numeric array=w5362) -> (sum=w5361:dbl)
              }
              n3302 = Select(t=w5348, s=w5349, f=w5347) -> (s? t:f=w5346:dbl)
              n3303 = Divide(x=w5353, y=w5346) -> (x/y=w5351:dbl[])
              n3304 = Bundle By Name(cluster=w5352, "magnitude"=w5351) -> (w5350:cluster{"f0":dbl, "df":dbl, "magnitude":dbl[]})
            }
          }
        }
        n3305 = case shown="True" w5292 {
          tunnel: w5293 -> [w5324 w5330]
          tunnel: [w5324 w5325] -> w5291
          frame False {
          }
          frame True {
            n3306 = Array Subset(array=w5330, index (row)=0 ("index"), length (row)=4 ("length"), index (col)=0 ("index"), length (col)=1 ("length")) -> (w5325:T66)
          }
        }
        n3307 = feedback-in #15(w5291) -> ()
        n3308 = Split 1D Array(array=w5305, index=2) -> (first subarray=→"FFT 1":cluster{"f0":dbl, "df":dbl, "magnitude":dbl[]}[], second subarray=→"FFT 2":cluster{"f0":dbl, "df":dbl, "magnitude":dbl[]}[])
      }
    }
    n3309 = local read "T2 calibration"() -> (w4247:T9)
    n3310 = local read "Offset Values"() -> (w4329:T20)
    n3311 = local read "T1 calibration"() -> (w4370:T9)
    n3312 = call-poly <vilib>:"Index Waveform Array.vi"("index"=16, "waveform array"=w4312) -> ("waveform"=w4346:waveform(dbl))  [unwired: 8 in, 1 out]
    n3313 = Unbundle By Name(w4361) -> ("Y"=w4369:dbl[])
    n3314 = Unbundle By Name(w4358) -> ("Y"=w4368:dbl[])
    n3315 = local read "Offset file step size"() -> (w4326:dbl)
    n3316 = Unbundle By Name(w4346) -> ("Y"=→"PSD Y Sum":dbl[])
    n3317 = call "calibrate trap data V2.vi"("Offset File step size"=w4326, "delta frequency"=w4328, "Dynamic offset update"="Dynamic offset\nupdate", "Offsets"=w4329, "T2 calibration"=w4247, "T2"=w4368, "T1 calibration"=w4370, "T1"=w4369) -> ("T2 force (pN)"=w4362:dbl[], "T2 position (nm)"=w4363:dbl[], "T1 force (pN)"=w4364:dbl[], "T1 position (nm)"=w4365:dbl[])
    n3318 = Bundle By Name(cluster=w4361, "Y"=w4365) -> (w4360:waveform(dbl))
    n3319 = Bundle By Name(cluster=w4361, "Y"=w4364) -> (w4359:waveform(dbl))
    n3320 = Bundle By Name(cluster=w4358, "Y"=w4363) -> (w4357:waveform(dbl))
    n3321 = Bundle By Name(cluster=w4358, "Y"=w4362) -> (w4356:waveform(dbl))
    n3322 = Subtract(x=w4365, y=w4363) -> (x-y=w4525:dbl[])
    n3323 = Negate(x=w4525) -> (-x=w4408:dbl[])
    n3324 = Subtract(x=w4408, y="Offset (nm)") -> (x-y=w4511:dbl[])
    n3325 = case "Choose calibrated display" shown="2" "Calibration" {
      tunnel: w4361 -> [w4938 _ _]
      tunnel: w4358 -> [w4937 _ _]
      tunnel: [w4938 w4940 w4942] -> w4341
      tunnel: [w4937 w4939 w4941] -> w4535
      tunnel: w4360 -> [_ w4940 _]
      tunnel: w4359 -> [_ _ w4942]
      tunnel: w4357 -> [_ w4939 _]
      tunnel: w4356 -> [_ _ w4941]
      frame 0, Default {
      }
      frame 1 {
      }
      frame 2 {
      }
    }
    n3326 = Bundle By Name(cluster=w4361, "Y"=w4511) -> (w4355:waveform(dbl))
    "Bead Separation" <- w4355
    n3327 = feedback #16(w4511) -> (w4510:dbl[])
    n3328 = Build Array (concatenate)(w4511, w4510) -> (w4366:dbl[])
    n3329 = Split 1D Array(array=w4366, index=w4264) -> (first subarray=w4367:dbl[])  [unwired: 1 out]
    n3330 = feedback-in #16(w4367) -> ()
    n3331 = Build Array(w4361, w4360, w4359, w4358, w4357, w4356, w4355) -> (w4354:waveform(dbl)[])
    n3332 = Not(x="Trap Trig. Fl.") -> (.not. x?=w4430:bool)
    n3333 = Unbundle By Name(w4341) -> ("Y"=w4409:dbl[])
    n3334 = Unbundle By Name(w4535) -> ("Y"=w4512:dbl[])
    n3335 = call-poly <vilib>:"Mean.vi"("X"=w4367) -> ("mean"=w4507:dbl)  [unwired: 1 out]
    "Bead Mean (nm)" <- w4507
    n3336 = Multiply(x=w4535, y=-1.0) -> (x*y=w4337:waveform(dbl))
    n3337 = call-poly <vilib>:"Mean.vi"("X"=w4409) -> ("mean"=w4412:dbl)  [unwired: 1 out]
    "T1 X" <- w4412
    n3338 = call-poly <vilib>:"Mean.vi"("X"=w4512) -> ("mean"=w4411:dbl)  [unwired: 1 out]
    "T2 X" <- w4411
    n3339 = Subtract(x=w4367, y=w4507) -> (x-y=w4506:dbl[])
    n3340 = Add(1:w4337, 2:w4341) -> (0:w4340:waveform(dbl))  [unwired: 1 in, 1 out]
    n3341 = Square(x=w4506) -> (x^2=w4505:dbl[])
    n3342 = Divide(x=w4340, y=2.0) -> (x/y=w4338:waveform(dbl))
    n3343 = Negate(x=w4512) -> (-x=w4378:dbl[])
    n3344 = call-poly <vilib>:"Mean.vi"("X"=w4505) -> ("mean"=w4504:dbl)  [unwired: 1 out]
    n3345 = Negate(x=w4411) -> (-x=w4410:dbl)
    n3346 = Square Root(x=w4504) -> (sqrt(x)=w4503:dbl)
    n3347 = Add(x=w4409, y=w4378) -> (x+y=w4513:dbl[])
    n3348 = Add(x=w4412, y=w4410) -> (x+y=w4531:dbl)
    n3349 = Multiply(x=10.0, y=w4503) -> (x*y=→"RMS (Ang)":dbl)
    n3350 = Divide(x=w4513, y=2.0) -> (x/y=w4381:dbl[])
    n3351 = Subtract(x=w4412, y=w4410) -> (x-y=→"Difference":dbl)
    n3352 = Build Array(w4341, w4337, w4338) -> (→"Force":waveform(dbl)[])
    n3353 = Select(t=w4378, s="Only check fixed trap T2", f=w4381) -> (s? t:f=→"Vec Mean of T1 T2":dbl[])
    n3354 = Divide(x=w4531, y=2.0) -> (x/y=w4323:dbl)
    "Mean" <- w4323
    n3355 = feedback-in #17("Trap Trig. Fl.") -> ()
    n3356 = feedback #17("Trap Trig. Fl.") -> (w4428:bool)
    n3357 = And(x=w4430, y=w4428) -> (x .and. y?=w4429:bool)
    n3358 = case "If have just turned off triggering" shown="True" w4429 {
      tunnel: w4334 -> [_ w4755]
      tunnel: w4424 -> [_ w4754]
      frame False {
      }
      frame True {
        w4753 = FALSE ("FPGA Trap Trig")
        n3359 = xnode "Read/Write Control"("FPGA VI Reference In"=w4755, "error in"=w4754, "FPGA Trap Trig"=w4753) -> ("FPGA VI Reference Out"=w4752:T41, "error out"=w4751:errorcluster)
        n3360 = xnode "Read/Write Control"("FPGA VI Reference In"=w4752, "error in"=w4751, "TTrig?"=w4753) -> ()  [unwired: 2 out]
        n3361 = local write "Initializing"(FALSE ("Initializing")) -> ()
        n3362 = local write "Triggered"(FALSE ("Triggered")) -> ()
        n3363 = local write "Waiting"(FALSE ("Waiting")) -> ()
      }
    }
    n3364 = Not(x=w4428) -> (.not. x?=w4441:bool)
    n3365 = And(x="Trap Trig. Fl.", y=w4441) -> (x .and. y?=w4438:bool)
    n3366 = Or(x=w4438, y="Reinitialize") -> (x .or. y?=w4427:bool)
    n3367 = feedback #18(w4434) -> (w4439:string)
    n3368 = Select(t=w4434, s=w4438, f=w4439) -> (s? t:f=w4433:string)
    n3369 = Select(t=w4434, s="Reinitialize", f=w4433) -> (s? t:f=w4432:string)
    n3370 = local read "Tether"() -> (w4515:bool)
    n3371 = feedback #19(0) -> (w4436:i32)
    n3372 = case "For determining if there is a tether still" shown="True" w4515 {
      tunnel: w4323 -> [_ w4864]
      frame False {
      }
      frame True {
        n3373 = Greater?(x="Lost Tether Alarm Threshold (pN)", y=w4864) -> (0:w4862:bool)
        n3374 = case shown="True" w4862 {
          frame False {
          }
          frame True {
            w4865 = FALSE ("Value (Signaling)")
            n3375 = flat-sequence {
              frame #0 {
                # "stop only if saving"
                n3376 = local read "Saving..."() -> (w4877:bool)
                n3377 = And(x=w4877, y="TA Cancel Save?") -> (x .and. y?=w4876:bool)
                n3378 = local write "Stop Saving"(w4876) -> ()
              }
              frame #1 {
                n3379 = case shown="True" "TA Green Off?" {
                  frame False {
                  }
                  frame True {
                    w4880 = FALSE ("Fl. Triggered...")
                    n3380 = local write "Fl. Triggered..."(w4880) -> ()
                    n3381 = property on="Green Laser ON" class="Bool (strict)"("Val(Sgnl)"=w4880) -> ()  [unwired: 2 in, 2 out]
                  }
                }
              }
            }
            n3382 = local read "Time tether formed"() -> (w4871:timestamp)
            n3383 = Get Date/Time In Seconds() -> (seconds since 1Jan1904=w4872:timestamp)
            n3384 = Subtract(x=w4872, y=w4871) -> (x-y=w4870:dbl)
            n3385 = Number To Decimal String(number=w4870) -> (decimal integer string=w4867:string)  [unwired: 1 out]
            n3386 = local read "Messages"() -> (w4874:string)
            n3387 = call <vilib>:"Beep.vi"() -> ()  [unwired: 3 in, 9 out]
            n3388 = Concatenate Strings("Lost tether (" ("Message to add"), w4867, " s)." ("string")) -> (w4869:string)
            n3389 = local write "Tether"(FALSE ("Tether")) -> ()
            n3390 = call "Update messages.vi"("Message to add"=w4869, "Old message string"=w4874) -> ("New message string"=w4873:string)
            n3391 = local write "Messages"(w4873) -> ()
            n3392 = property on="Fl. Triggered..." class="Bool (strict)"("Val(Sgnl)"=w4865) -> ()  [unwired: 2 in, 2 out]
            n3393 = local write "Dip for Protein"(w4865) -> ()
            n3394 = property on="Trap Pos. FB ON" class="Bool (strict)"("Val(Sgnl)"=w4865) -> ()  [unwired: 2 in, 2 out]
            n3395 = property on="Trap Trig. Fl." class="Bool (strict)"("Val(Sgnl)"=w4865) -> ()  [unwired: 2 in, 2 out]
          }
        }
      }
    }
    n3396 = case "For triggering actions based on the trap position (e.g., turning the excitation laser on if trap under feedback moves so far)" shown="True" "Trap Trig. Fl." {
      tunnel: w4257 -> [_ w4768]
      tunnel: w4432 -> [_ w4767]
      tunnel: ["" ("t") w4766] -> w4440
      tunnel: w4427 -> [_ w4765]
      tunnel: [0 ("t") w4764] -> w4437
      tunnel: w4436 -> [_ w4763]
      tunnel: w4334 -> [_ w4762]
      tunnel: w4424 -> [_ w4761]
      frame False {
      }
      frame True {
        n3397 = case shown="\"Wait for trigger\"" w4767 {
          tunnel: w4768 -> [w4785 _ _ w4833]
          tunnel: [w4782 w4814 "" ("t") w4836] -> w4766
          tunnel: w4765 -> [_ _ _ w4824]
          tunnel: [w4781 w4811 0 ("t") w4825] -> w4764
          tunnel: w4763 -> [_ w4813 _ w4831]
          tunnel: w4762 -> [w4770 w4808 _ w4827]
          tunnel: w4761 -> [w4769 w4807 _ w4826]
          frame "Wait for trigger" {
            n3398 = local read "Trap Trig. (FPGA)"() -> (w4773:bool)
            n3399 = Subtract(x=w4785, y="Mean T1 Position\nto compare (nm)") -> (x-y=w4778:dbl[])
            n3400 = call <vilib>:"Std Deviation and Variance.vi"("X"=w4778) -> ("mean"=→"mean":dbl, "standard deviation"=→"standard\ndeviation":dbl)  [unwired: 1 in, 1 out]
            n3401 = Array Max & Min(array=w4778) -> (max value=→"max value":dbl, min value=→"min value":dbl)  [unwired: 2 out]
            n3402 = Greater?(x=w4778, y="Threshold (nm)") -> (0:w4788:bool[])
            n3403 = case shown="True" w4773 {
              tunnel: w4770 -> [_ w4794]
              tunnel: w4769 -> [_ w4793]
              tunnel: [FALSE ("TTrig?") w4792] -> w4776
              frame False {
              }
              frame True {
                n3404 = xnode "Read/Write Control"("FPGA VI Reference In"=w4794, "error in"=w4793) -> ("TTrig?"=w4792:bool)  [unwired: 2 out]
              }
            }
            n3405 = Or Array Elements(Boolean array=w4788) -> (logical OR=w4775:bool)
            n3406 = Select(t=w4776, s=w4773, f=w4775) -> (s? t:f=w4774:bool)
            n3407 = Not(x=w4773) -> (.not. x?=w4772:bool)
            n3408 = And(x=w4774, y=w4772) -> (x .and. y?=w4771:bool)
            n3409 = Select(t="Triggered", s=w4774, f="Wait for trigger") -> (s? t:f=w4782:string)
            n3410 = case shown="True" w4774 {
              tunnel: [0 0] -> w4781
              tunnel: w4770 -> [_ w4799]
              tunnel: w4769 -> [_ w4798]
              frame False {
                "Waiting" <- TRUE ("Waiting")
              }
              frame True {
                n3411 = xnode "Read/Write Control"("FPGA VI Reference In"=w4799, "error in"=w4798, "TTrig?"=FALSE) -> ()  [unwired: 2 out]
                n3412 = local read "Messages"() -> (w4802:string)
                n3413 = call <vilib>:"Beep.vi"() -> ()  [unwired: 12 in]
                n3414 = call "Update messages.vi"("Message to add"="Unwinding trigger.", "Old message string"=w4802) -> ("New message string"=w4803:string)
                n3415 = local write "Messages"(w4803) -> ()
                n3416 = local write "Waiting"(FALSE ("Waiting")) -> ()
                "Triggered" <- TRUE ("Triggered")
              }
            }
            n3417 = case "Only need to turn on laser if host triggered" shown="True" w4771 {
              frame False {
              }
              frame True {
                n3418 = property on="Green Laser ON" class="Bool (strict)"("Val(Sgnl)"=TRUE ("Value (Signaling)")) -> ()  [unwired: 2 in, 2 out]
              }
            }
          }
          frame "Triggered" {
            n3419 = local read "Trap Trig. (FPGA)"() -> (w4810:bool)
            n3420 = Increment(x=w4813) -> (x+1=w4811:i32)
            n3421 = Greater Or Equal?(x=w4811, y="Fl. ON time (n)") -> (x >= y?=w4809:bool)
            n3422 = Select(t="Wait for trigger", s=w4809, f="Triggered" ("t")) -> (s? t:f=w4814:string)
            n3423 = And(x=w4809, y=w4810) -> (x .and. y?=w4806:bool)
            n3424 = case shown="True" w4806 {
              tunnel: w4808 -> [_ w4818]
              tunnel: w4807 -> [_ w4817]
              frame False {
              }
              frame True {
                n3425 = xnode "Read/Write Control"("FPGA VI Reference In"=w4818, "error in"=w4817, "FPGA Trap Trig"=TRUE) -> ()  [unwired: 2 out]
              }
            }
            n3426 = case shown="True" w4809 {
              frame False {
              }
              frame True {
                w4820 = FALSE ("Value (Signaling)")
                n3427 = local write "Triggered"(w4820) -> ()
                n3428 = local write "Waiting"(TRUE ("Waiting")) -> ()
                n3429 = property on="Green Laser ON" class="Bool (strict)"("Val(Sgnl)"=w4820) -> ()  [unwired: 2 in, 2 out]